vi "MH.vi"() -> ()   [LabVIEW 2018]
uses:
  <vilib>/Utility/file.llb/Read Delimited Spreadsheet (DBL).vi
panel:
  in  "stop":bool
  in  "Main Tab Control":T1(tab)
  in  "?":bool
  in  "MH data folder:":path=path "C:/Research/data/MH"
  out "File path for today's data":path
  in  "Short comment on today's measurement (will be the info file filename)":string="todayssample"
  in  "Long comment on today's measurement":string="This is where you can put more information about this measurement."
  in  "ImpedanceGFactor Tab Control":enum32{"H-Coil", "M- Coil"}(tab)
  in  "H-Coil Tab Control":T2(tab)
  in  "H-Coil VNA Control Tab Control":enum32{"Control Panel", "Display Panel"}(tab)
  out "isFileWritten? 2":string
  out "writeImpeadanceDataError 2":errorcluster
  in  "writeImpeadanceDataFunctionName":string
  out "Data file: data 3":dbl[][](array[numeric])
  in  "vnaEndFreq":dbl=30000000.0
  in  "vnaStartFreq":dbl=100000.0
  in  "vnaNumOfRecordings":dbl=5001.0
  in  "vnaFunctionName":string="vnaRead"
  in  "vnaRead":path=path "C:/Research/MH program/tempsScopeAndVNALabview.py"
  in  "H coil impedance data source:":enum32{"Measure:", "From data file:"}(radio)
  in  "Path: Hcoil data 2":path=path "C:/Research/data/RohdeZND/20180620/20180620-Hcoil.csv"
  in  "?":bool
  out "Data file: data 2":dbl[][](array[numeric])
  out "vnaErrorOut":errorcluster
  out "Impedance (Magnitude)":cluster{dbl[], dbl[]}(graph)
  out "Impedance (Phase)":cluster{dbl[], dbl[]}(graph)
  in  "H-Coil Manual Fit Control Tab Control":enum32{"Control Tab", "Display Tab"}(tab)
  in  "numf 1H":i16=1000
  in  "fmax 1H":dbl=20000000.0
  in  "f0 1H":dbl=1.0
  in  "Num of components in BNC model 1H":i16=10
  in  "Input: BNC cable length (ft) 1H":dbl=4.0 format="%#_6f"
  in  "Input: R2 (Ohms) 1H":dbl=10.0 format="%#_6f"
  in  "Input: R1 (Ohms) 1H":dbl=14.6 format="%#_6f"
  in  "Input: L (nH) 1H":dbl=3000.0 format="%#_6f"
  in  "Input: C (pF) 1H":dbl=60.0 format="%#_6f"
  in  "Input: C (pF) 2H":dbl=70.0 format="%#_6f"
  in  "Input: L (nH) 2H":dbl=800.0 format="%#_6f"
  in  "Input: R1 (Ohms) 2H":dbl=11.0 format="%#_6f"
  in  "Input: R2 (Ohms) 2H":dbl=25.0 format="%#_6f"
  in  "Input: BNC cable length (ft) 2H":dbl=4.0 format="%#_6f"
  in  "Num of components in BNC model 2H":i16=4
  in  "f0 2H":dbl=1.0
  in  "fmax 2H":dbl=40000000.0
  in  "numf 2H":i16=1000
  in  "?":bool
  out "Simulation 2: error out 2":errorcluster
  out "Simulation 1: error out":errorcluster
  out "Simulation 1: data":dbl[][](array[numeric]) format="%#_6f"
  out "Simulation 2: data":dbl[][](array[numeric]) format="%#_6f"
  in  "module path":path=path "C:/Research/MH program/impedancesim.py"
  in  "function name":string="impedance"
  out "?":string
  out "?":string
  out "?":string
  in  "?":bool
  in  "?":bool
  in  "?":bool=TRUE
  out "Impedance (phase)":cluster{"array":dbl[], "array":dbl[]}[](graph)
  out "Impedance (magnitude)":cluster{"array":dbl[], "array":dbl[]}[](graph)
  out "Impedance (magnitude) (zoomed)":T3(graph)
  out "Impedance (phase) (zoomed)":T3(graph)
  in  "H-Coil Automatic Fit Control Tab Control":enum32{"Control Panel", "Display Panel"}(tab)
  out "fit parameters":dbl[](array[numeric])
  in  "Vary numlumps?\n(Choose False)":string="False"
  in  "Vary BNClen?\n(Choose False)":string="False"
  in  "Vary R2?":string="True"
  in  "Vary R1?":string="False"
  in  "Vary L?":string="True"
  in  "Vary C?":string="True"
  out "BNC length (ft) H":dbl=4.0 format="%#_6f"
  out "Num of components in BNC model fit H":i16=4
  out "R20 (Ohms) H":dbl=25.0 format="%#_6f"
  out "R10 (Ohms) H":dbl=11.0 format="%#_6f"
  out "Initial value:\nL0 (H) H":dbl=800.0 format="%#_6e"
  out "C0 (F) H":dbl=70.0 format="%#_6e"
  in  "?":bool
  out "Simulation 1: error out 3":errorcluster
  in  "module path impedance fit":path=path "C:/Research/MH program/impedancelmfitforlv.py"
  in  "function name impedance fit":string="impedancelmfit"
  out "return value gH 2":dbl[][](array[numeric])
  out "cluster":T4
  out "Impedance data":cluster{dbl[], dbl[], dbl[]}
  in  "Start data pt":i32=2
  out "Total data points":i32
  in  "End data point":i32=3000
  out "Impedance mag near zero:\nFit vs data":cluster{dbl[], dbl[]}[](graph)
  out "Impedance mag data near zero: Use this to find R1":cluster{dbl[], dbl[]}(graph)
  out "?":string
  out "Impedance phase 2":T3(graph)
  out "Impedance magnitude (Ohms) 2":T3(graph)
  in  "H-Coil GFactor Control Tab Control":enum32{"Control Panel", "Display Panel"}(tab)
  in  "Coil 2":string="Hcoil"
  in  "Coil parameter source (if calculating g-factor)":enum32{"Simulation", "Fit"}(radio)=enum."Fit"
  in  "Rosc":dbl=1000000.0 format="%#_13g"
  in  "start gH":bool
  out "numf gH":i16=1000
  out "fmax gH":dbl=40000000.0
  out "f0 gH":dbl=1.0
  out "Num of components in BNC model gH":i16=4
  out "Input: BNC cable length (ft) gH":dbl=4.0 format="%#_6f"
  out "Input: R2 (Ohms) gH":dbl=25.0 format="%#_6f"
  out "Input: R1 (Ohms) gH":dbl=11.0 format="%#_6f"
  out "Input: L (H) gH":dbl=800.0 format="%#_6f"
  out "Input: C (F) gH":dbl=70.0 format="%#_6f"
  out "numf gH 2":i16=1000
  out "fmax gH 2":dbl=40000000.0
  out "f0 gH 2":dbl=1.0
  out "Num of components in BNC model gH 2":i16=4
  out "Input: BNC cable length (ft) gH 2":dbl=4.0 format="%#_6f"
  out "Input: R2 (Ohms) gH 2":dbl=25.0 format="%#_6f"
  out "Input: R1 (Ohms) gH 2":dbl=11.0 format="%#_6f"
  out "Input: L (H) gH 2":dbl=800.0 format="%#_6f"
  out "Input: C (F) gH 2":dbl=70.0 format="%#_6f"
  in  "G-Factor Calculation":T5(radio)
  in  "Date 3":string
  in  "Time 3":string
  in  "Filepath Name":string="C:/Research/Data/MH"
  out "readG-FactorFilesError":errorcluster
  in  "ReadDataFunctionName":string="readGFactorData"
  out "Simulation 1: error out 2":errorcluster
  out "return value gH":dbl[][](array[numeric])
  in  "function name gfactor":string="gfactor"
  in  "module path g-factor":path=path "C:/Research/MH program/gfactor.py"
  out "gfactor H (phase)":T6(graph)
  out "gfactor H (magnitude)":T6(graph)
  in  "M-Coil Control Tab Control":T7(tab)
  in  "M-Coil VNA Control Tab Control":enum32{"Control Panel", "Display Panel"}(tab)
  in  "writeImpeadanceDataFunctionName 2":string
  out "writeImpeadanceDataError":errorcluster
  out "isFileWritten?":string
  out "Data file: data 4":dbl[][](array[numeric])
  out "Data file: M coil data":dbl[][](array[numeric])
  in  "Path: Mcoil data":path=path "C:/Research/data/RohdeZND/20180621/20180621-Mcoil.csv"
  out "error out":errorcluster
  in  "M coil impedance data source:":enum32{"Measure:", "From data file:"}(radio)
  in  "?":bool
  in  "vnaRead 2":path=path "C:/Research/MH program/tempsScopeAndVNALabview.py"
  in  "vnaFunctionName 2":string="vnaRead"
  in  "vnaNumOfRecordings 2":dbl=5001.0
  in  "vnaStartFreq 2":dbl=100000.0
  in  "vnaEndFreq 2":dbl=30000000.0
  out "M Impedance (Phase)":cluster{dbl[], dbl[]}(graph)
  out "M Impedance (Magnitude)":cluster{dbl[], dbl[]}(graph)
  in  "M-Coil Manual Fit Control Tab Control":enum32{"Control Panel", "Display Panel"}(tab)
  in  "numf 1M":i16=1000
  in  "fmax 1M":dbl=40000000.0
  in  "f0 1M":dbl=1.0
  in  "Num of components in BNC model 1M":i16=10
  in  "Input: BNC cable length (ft) 1M":dbl=4.0 format="%#_6f"
  in  "Input: R2 (Ohms) 1M":dbl=14.5 format="%#_6f"
  in  "Input: R1 (Ohms) 1M":dbl=8.05 format="%#_6f"
  in  "Input: L (nH) 1M":dbl=1400.0 format="%#_6f"
  in  "Input: C (pF) 1M":dbl=64.0 format="%#_6f"
  in  "Input: C (pF) 2M":dbl=70.0 format="%#_6f"
  in  "Input: L (nH) 2M":dbl=800.0 format="%#_6f"
  in  "Input: R1 (Ohms) 2M":dbl=11.0 format="%#_6f"
  in  "Input: R2 (Ohms) 2M":dbl=25.0 format="%#_6f"
  in  "Input: BNC cable length (ft) 2M":dbl=4.0 format="%#_6f"
  in  "Num of components in BNC model 2M":i16=4
  in  "f0 2M":dbl=1.0
  in  "fmax 2M":dbl=40000000.0
  in  "numf 2M":i16=1000
  in  "python impedance":path=path "C:/Research/MH program/impedancesim.py"
  in  "python impedance function name":string="impedance"
  in  "?":bool
  out "Simulation 2M: data":dbl[][](array[numeric]) format="%#_6f"
  out "Simulation 1M: data":dbl[][](array[numeric]) format="%#_6f"
  out "Simulation 1M: error out":errorcluster
  out "Simulation 2M: error out":errorcluster
  out "?":string
  out "?":string
  out "?":string
  in  "?":bool
  in  "?":bool
  in  "?":bool=TRUE
  out "Impedance (phase) M":cluster{"array":dbl[], "array":dbl[]}[](graph)
  out "Impedance (magnitude) M":cluster{"array":dbl[], "array":dbl[]}[](graph)
  out "Impedance (magnitude) M (zoomed)":T3(graph)
  out "Impedance (phase) M (zoomed)":T3(graph)
  in  "M-Coil Automatic Fit Control Tab Control":enum32{"Control Panel", "Display Panel"}(tab)
  out "C0 (F) H 2":dbl=70.0 format="%#_6e"
  out "Initial value:\nL0 (H) H 2":dbl=800.0 format="%#_6e"
  out "R10 (Ohms) H 2":dbl=11.0 format="%#_6f"
  out "R20 (Ohms) H 2":dbl=25.0 format="%#_6f"
  out "Num of components in BNC model fit H 2":i16=4
  out "BNC length (ft) H 2":dbl=4.0 format="%#_6f"
  in  "Vary C? 2":string="True"
  in  "Vary L? 2":string="True"
  in  "Vary R1? 2":string="False"
  in  "Vary R2? 2":string="True"
  in  "Vary BNClen?\n(Choose False) 2":string="False"
  in  "Vary numlumps?\n(Choose False) 2":string="False"
  in  "?":bool
  in  "End data point 2":i32=3000
  out "Total data points 2":i32
  out "Impedance data 2":cluster{dbl[], dbl[], dbl[]}
  in  "Start data pt 2":i32=2
  out "Simulation 1: error out 4":errorcluster
  in  "module path impedance fit 2":path=path "C:/Research/MH program/impedancelmfitforlv.py"
  in  "function name impedance fit 2":string="impedancelmfit"
  out "return value":dbl[][](array[numeric])
  out "fit parameters 2":dbl[](array[numeric])
  out "cluster 2":T4
  out "Impedance magnitude (Ohms)":T3(graph)
  out "Impedance phase":T3(graph)
  out "Impedance mag near zero:\nFit vs data 2":cluster{dbl[], dbl[]}[](graph)
  out "Impedance mag near zero: Use this to find R1":cluster{dbl[], dbl[]}(graph)
  in  "M-Coil GFactor Control Tab Control":enum32{"Control Panel", "Display Panel"}(tab)
  in  "Coil":string="Mcoil"
  in  "Filepath Name 2":string="C:/Research/Data/MH"
  in  "Time 2":string
  in  "Date 2":string
  in  "Rosc 2":dbl=1000000.0 format="%#_13g"
  in  "G-Factor Calculation 2":T5(radio)
  in  "Coil parameter source":enum32{"Simulation", "Fit"}(radio)=enum."Fit"
  in  "start gM":bool
  out "Input: C (F) gM":dbl=70.0 format="%#_6f"
  out "Input: L (H) gM":dbl=800.0 format="%#_6f"
  out "Input: R1 (Ohms) gM":dbl=11.0 format="%#_6f"
  out "Input: R2 (Ohms) gM":dbl=25.0 format="%#_6f"
  out "Num of components in BNC model gM":i16=4
  out "Input: BNC cable length (ft) gM":dbl=4.0 format="%#_6f"
  out "f0 gM":dbl=1.0
  out "fmax gM":dbl=40000000.0
  out "numf gM":i16=1000
  out "numf gM 2":i16=1000
  out "fmax gM 2":dbl=40000000.0
  out "f0 gM 2":dbl=1.0
  out "Num of components in BNC model gM 2":i16=4
  out "Input: BNC cable length (ft) gM 2":dbl=4.0 format="%#_6f"
  out "Input: R2 (Ohms) gM 2":dbl=25.0 format="%#_6f"
  out "Input: R1 (Ohms) gM 2":dbl=11.0 format="%#_6f"
  out "Input: L (H) gM 2":dbl=800.0 format="%#_6f"
  out "Input: C (F) gM 2":dbl=70.0 format="%#_6f"
  in  "ReadDataFunctionName 2":string="readGFactorData"
  in  "module path g-factor 2":path=path "C:/Research/MH program/gfactor.py"
  in  "function name gfactor 2":string="gfactor"
  out "readG-FactorFilesError  2":errorcluster
  out "gfactor M: error out":errorcluster
  out "return value gM":dbl[][](array[numeric])
  out "gfactor M (magnitude)":T6(graph)
  out "gfactor M (phase)":T6(graph)
  in  "VoltageTemp Control Tab Control":enum32{"Control Panel", "Display Panel"}(tab)
  in  "Run with Simulator":bool=TRUE
  in  "Run":i64
  in  "Run":dbl
  in  "readDataFileVoltageName":string="readVoltageData"
  in  "Voltage data source:":enum32{"Measure:", "From data file:"}(radio)
  in  "readDataFileTemperatureName":string="readTempData"
  in  "Date":string
  in  "Time":string
  in  "numChan 2":i32=2
  in  "dataFilePath":string="C:\\Research\\data\\MH"
  in  "?":bool
  in  "numChan":i32=2
  in  "scopeNumCollects":i32=3
  in  "shortRecordLength":i32=10000
  in  "longRecordLength 2":i32=100000
  in  "mainForAmbrell":string="mainForAmbrell"
  in  "ModulePath":path=path "C:/Research/SenaCodeBaseandDocuments/CodeBaseRepo/SummerResearch2019CodeBase/MH program/tempsScopeAndVNALabviewMHProgram.py"
  in  "Operating Frequency of EASYHEAT":dbl=227000.0
  in  "Run Checkscale?":bool=TRUE
  out "readDataFileTempError":errorcluster
  out "readDataFileVoltageError":errorcluster
  out "mainForAmbrellError":errorcluster
  out "Oscilloscope Channel 1 Output Graph":cluster{dbl[], dbl[]}[](graph)
  out "Oscilloscope Channel 2 Output Graph":cluster{dbl[], dbl[]}[](graph)
  out "Opsens Channel 1":cluster{"Array 2":dbl[], "Array 3":dbl[]}[](graph)
  # "Instructions for making an M(H) measurement"
  # "0. (Rarely) Calibrate H (still need to work on this)\n1. (Sometimes) Measure impedance of H coil using vector network analyzer (Sena's program) or load from file\n2. (Sometimes) Model impedance of H coil to find coil parameters (Zoe's program)\n3. (Sometimes) Calculate g-factor of H coil (Zoe's program)\n4. (Sometimes) Measure impedance of M coil using vector network analyzer (Sena's program) or load from file\n5. (Sometimes) Model impedance of M coil to find coil parameters (Zoe's program)\n6. (Sometimes) Calculate g-factor of M coil (Zoe's program)\n7. (Every time) Center M coil by hand (no program)\n8. (Every time) Measure sample data - induced voltage using oscilloscope and temperature using opsens (Sena's program) or load from file(s)\n9. (Every time) Select voltage data to analyze (Emily's program)\n10. (Every time) Analyze voltage data to find M(H) for each run (Emily's program)\n11. (Every time) Save data (Emily's program)"
  # "CONNECT M COIL TO VNA!"
  # "H coil"
  # "Impedance\nsimulation 1\nparameters"
  # "Impedance\nsimulation 2\nparameters"
  # "Data file\nlocation"
  # "What to plot:"
  # "(toggle buttons below)"
  # "Simulation 1"
  # "Simulation 2"
  # "Data file"
  # "Values to initialize fit:"
  # "THIS MAY TAKE A\nCOUPLE MINUTES!"
  # "f"
  # "Z (mag)"
  # "Z (phase)"
  # "H coil"
  # "Calculate g-factor"
  # "Oscillosope\nimpedance:"
  # "THIS MAY TAKE A\nCOUPLE MINUTES!"
  # "Read Data File Controls"
  # "Impedance\nsimulation 1\nparameters"
  # "Fit\nparameters"
  # "CONNECT H COIL TO VNA!"
  # "M coil"
  # "Impedance\nsimulation 1\nparameters"
  # "Impedance\nsimulation 2\nparameters"
  # "Data file\nlocation"
  # "What to plot:"
  # "(toggle buttons below)"
  # "Simulation 1"
  # "Simulation 2"
  # "Data file"
  # "THIS MAY TAKE A\nCOUPLE MINUTES!"
  # "Read Data File Controls"
  # "M coil"
  # "Calculate g-factor"
  # "THIS MAY TAKE A\nCOUPLE MINUTES!"
  # "Oscillosope\nimpedance:"
  # "Impedance\nsimulation 1\nparameters"
  # "(Imported from\n last panel)"
  # "(Currently not working - need to decide on a data format)"
  # "Save data to an Excel file. Use multiple worksheets within one file to store the various types of data. e.g.\n-One worksheet to store basic info about the data collection and analysis:\n       -Date and time\n       -Calibration factors\n-One worksheet to store the Hcoil impedance\n       -Headers: Frequency (Hz) // Real component (Ohms) // Imag component (Ohms) // Note: Data from file or measured?\n       -freq, real, imag columns\n-One worksheet to store info on the Hcoil impedance model\n       -Was the impedance model the result of a manual fit (simulation) or an automatic fit?\n       -If automatic fit, which parameters were allowed to vary, and which were kept fixed?\n       -Values for C, L, R1, R2, BNClen, numlumps\n-One worksheet for Hcoil impedance model, similar to data\n       -Headers: Frequency (Hz) // Real component (Ohms) // Imag component (Ohms)\n       -freq, real, imag columns\n-One sheet showing a chart of impedance data vs model\n-One worksheet for Hcoil gfactor\n       -Headers: Frequency (Hz) // Real component  // Imag component \n       -freq, real, imag columns\n-One sheet showing a chart of Hcoil gfactor\n-Same series of sheets as above but for Mcoil\n-One worksheet to store basic info about the voltage/temperature data collection and analysis\n       -How many data collections? Record length?\n       -Time data collection was begun\n       -Info about temperature collection - time between data points?\n-One worksheet for EACH set of voltage data\n-One worksheet for temperature vs time data\n-One worksheet for all the M(H) curves analyzed\n-One sheet at the end showing a chart of M(H) for all data sets\n\n\nOpen question:\nIs it a good idea to do all this in Excel?? We could run into problems with memory for large Excel files. If Excel is a problem, a series of .txt or .csv files (one for each sheet above) could accomplish the same goals.\nIf we do it this way, we should create organized folders for each analysis."
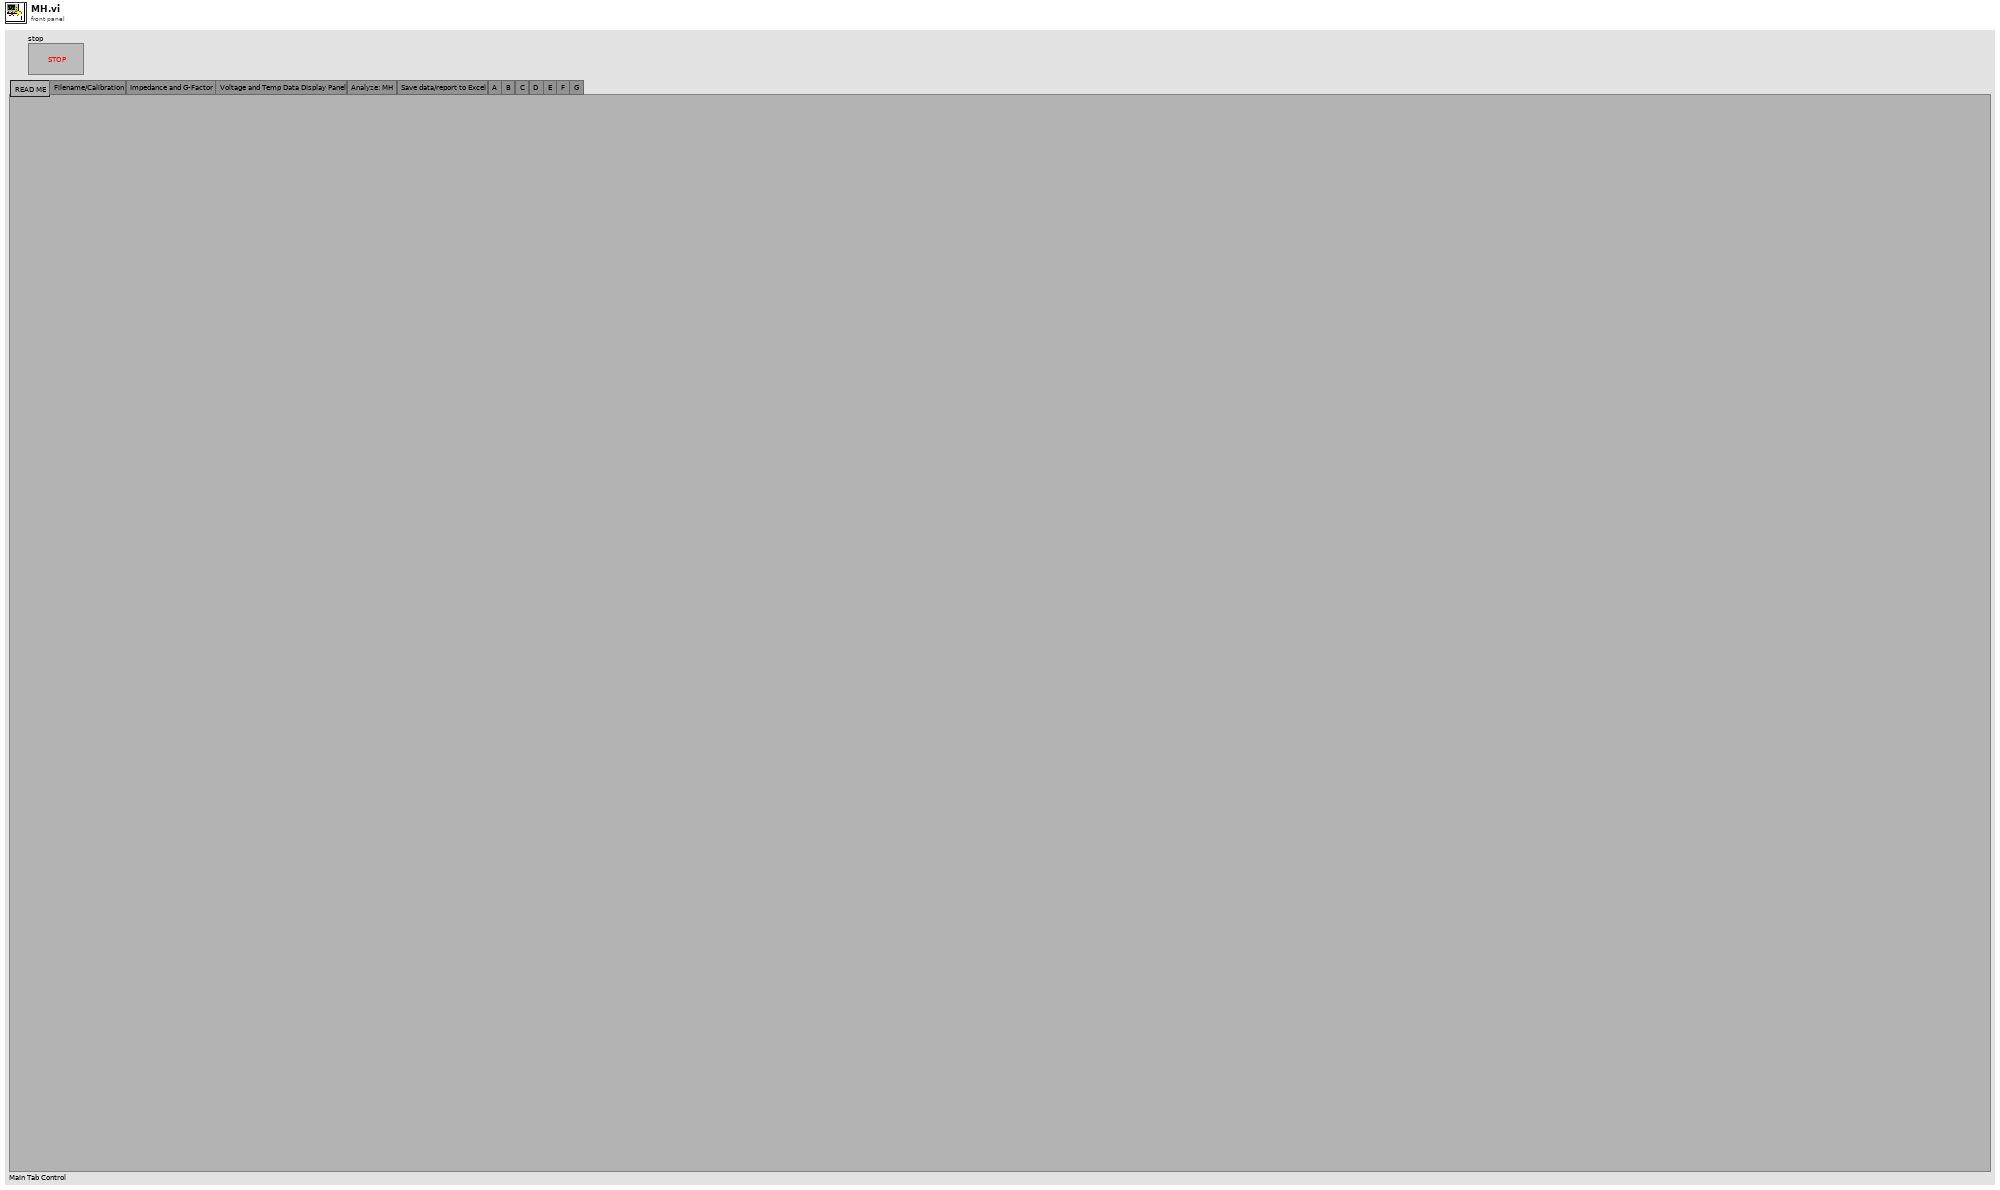
[diagram p1: front panel]
types:
  T1 = enum32{"READ ME", "Filename/Calibration", "Impedance and G-Factor", "Voltage and Temp Data Display Panel", "Analyze: MH", "Save data/report to Excel", "A", "B", "C", "D", "E", "F", "G"}
  T2 = enum32{"Get Impedance from VNA", "Manual Fit H-Coil", "Automatic Fit H-Coil", "G-Factor Calculation"}
  T3 = cluster{"return value 3":dbl[], "return value 3":dbl[]}[]
  T4 = cluster{"[0]":dbl, "[1]":dbl, "[2]":dbl, "[3]":dbl, "[4]":dbl, "[5]":dbl, "[6]":dbl, "[7]":dbl, "[8]":dbl}
  T5 = enum32{"Read data from a g-factor file", "Calculate G-factor"}
  T6 = cluster{"return value 3":dbl[], "return value 3":dbl[]}
  T7 = enum32{"Get Impedance from VNA", "Manual Fit M-Coil", "Automatic Fit M-Coil", "G-Factor Calculation"}
  T8 = cluster{dbl, dbl, "Input: R1 (Ohms) 1H":dbl, "Input: R2 (Ohms) 1H":dbl, "Input: BNC cable length (ft) 1H":dbl, "Num of components in BNC model 1H":i16, "f0 1H":dbl, "fmax 1H":dbl, "numf 1H":i16}
  T9 = cluster{dbl, dbl, "Input: R1 (Ohms) 2H":dbl, "Input: R2 (Ohms) 2H":dbl, "Input: BNC cable length (ft) 2H":dbl, "Num of components in BNC model 2H":i16, "f0 2H":dbl, "fmax 2H":dbl, "numf 2H":i16}
  T10 = cluster{dbl, dbl, "Input: R1 (Ohms) 2M":dbl, "Input: R2 (Ohms) 2M":dbl, "Input: BNC cable length (ft) 2M":dbl, "Num of components in BNC model 2M":i16, "f0 2M":dbl, "fmax 2M":dbl, "numf 2M":i16}
  T11 = cluster{dbl, dbl, "Input: R1 (Ohms) 1M":dbl, "Input: R2 (Ohms) 1M":dbl, "Input: BNC cable length (ft) 1M":dbl, "Num of components in BNC model 1M":i16, "f0 1M":dbl, "fmax 1M":dbl, "numf 1M":i16}
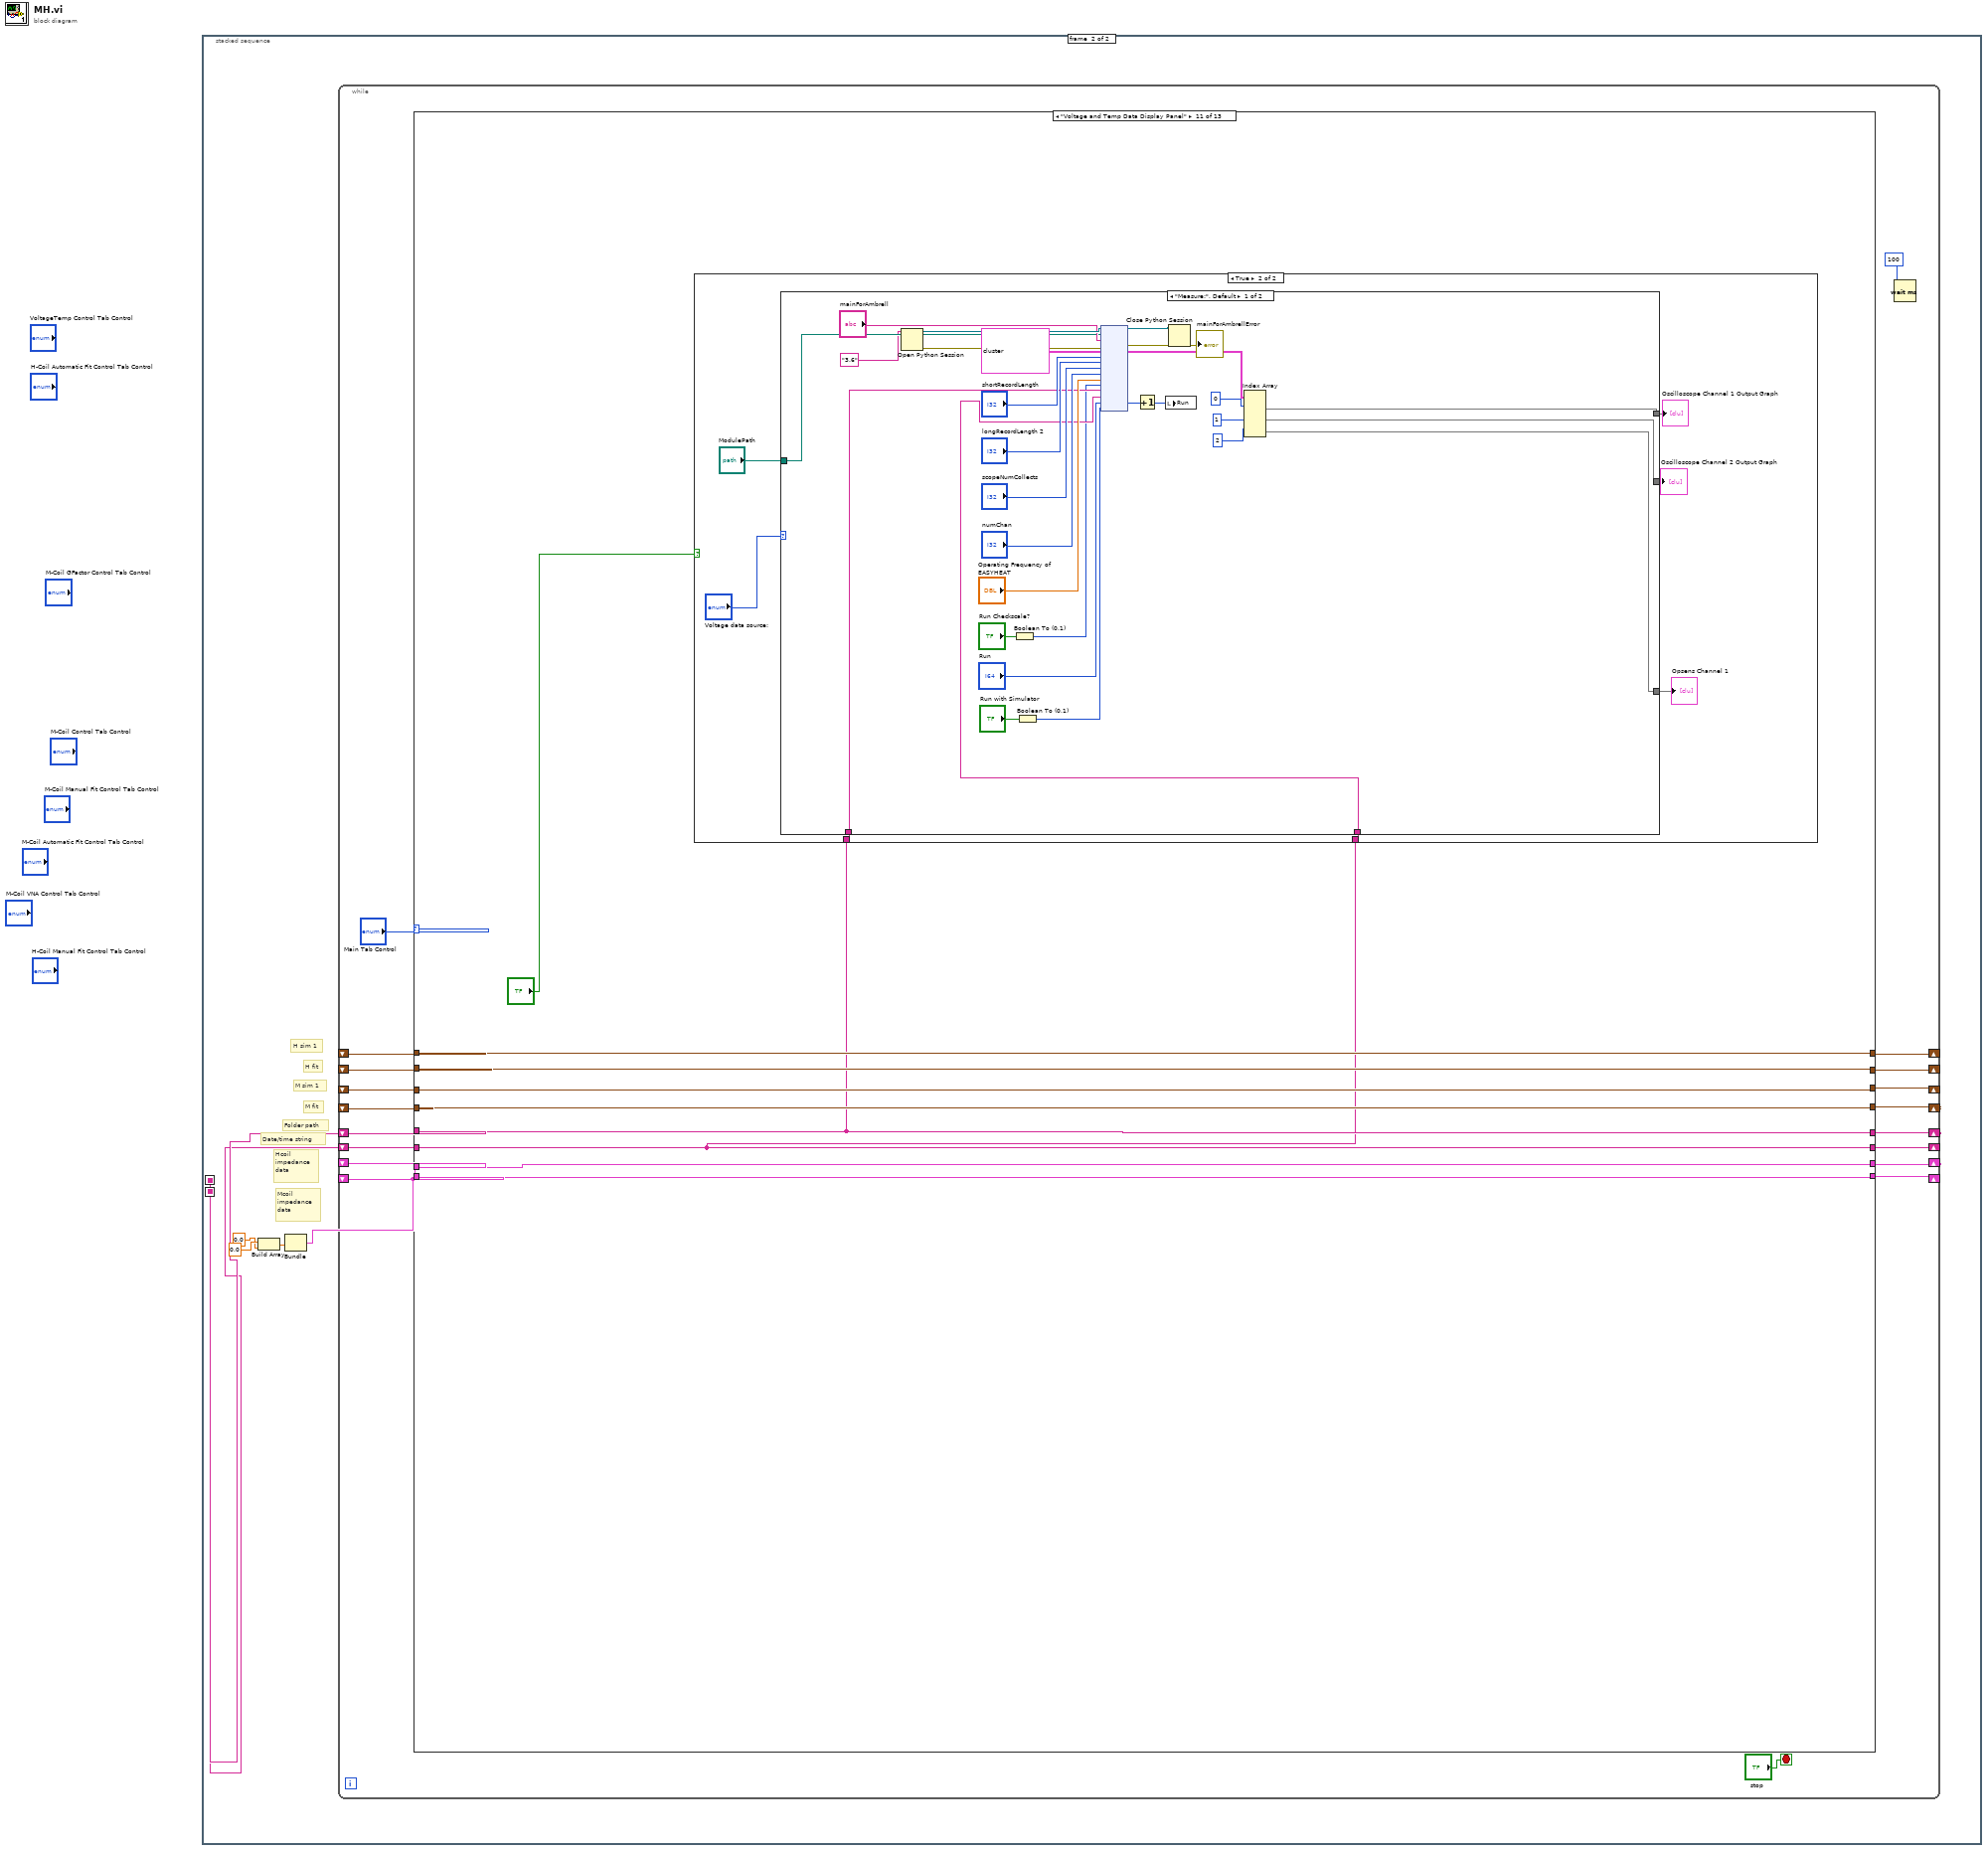
[diagram p0: block diagram]
diagram:
  n1 = stacked-sequence {
    seq-local: [w2 _] -> [_ w36]
    seq-local: [w1 _] -> [_ w35]
    frame #0 {
      n2 = stacked-sequence {
        seq-local: [w3 _ _] -> [_ w12 w14]
        tunnel: [_ w12 _] -> w2
        tunnel: [w4 _ _] -> w1
        frame #0 {
          w7 = "\\\\"
          n3 = Format Date/Time String(time format string (%c)="%Y%m%d") -> (date/time string=w6:string)  [unwired: 2 in]
          n4 = Format Date/Time String(time format string (%c)="%H%M%S") -> (date/time string=w5:string)  [unwired: 2 in]
          n5 = Path To String(path="MH data folder:") -> (string=w9:string)
          n6 = Concatenate Strings(w9, w7, w6, w7, w5) -> (w3:string)
          n7 = Concatenate Strings(w6, w5) -> (w4:string)
        }
        frame #1 {
          n8 = String To Path(string=w12) -> (path=w13:path)
          "File path for today's data" <- w13
          n9 = Create Folder(path (use dialog)=w13) -> ()  [unwired: 2 in, 3 out]
        }
        frame #2 {
          n10 = Concatenate Strings(w14, "\\\\", "Oscilloscope") -> (w25:string)
          n11 = Concatenate Strings(w14, "\\\\", "Opsens") -> (w21:string)
          n12 = Concatenate Strings(w14, "\\\\", "MHanalyzed") -> (w17:string)
          n13 = Concatenate Strings(w14, "\\\\", "Mcoil") -> (w29:string)
          n14 = Concatenate Strings(w14, "\\\\", "Hcoil") -> (w32:string)
          n15 = String To Path(string=w25) -> (path=w23:path)
          n16 = String To Path(string=w21) -> (path=w19:path)
          n17 = String To Path(string=w17) -> (path=w15:path)
          n18 = String To Path(string=w29) -> (path=w28:path)
          n19 = String To Path(string=w32) -> (path=w31:path)
          n20 = Create Folder(path (use dialog)=w23) -> ()  [unwired: 2 in, 3 out]
          n21 = Create Folder(path (use dialog)=w19) -> ()  [unwired: 2 in, 3 out]
          n22 = Create Folder(path (use dialog)=w15) -> ()  [unwired: 2 in, 3 out]
          n23 = Create Folder(path (use dialog)=w28) -> ()  [unwired: 2 in, 3 out]
          n24 = Create Folder(path (use dialog)=w31) -> ()  [unwired: 2 in, 3 out]
        }
      }
    }
    frame #1 {
      # "Date/time string"
      # "Folder path"
      # "H sim 1"
      # "H fit"
      # "M sim 1"
      # "M fit"
      # "Hcoil\nimpedance\ndata"
      # "Mcoil\nimpedance\ndata"
      n25 = Build Array(0.0, 0.0) -> (w37:dbl[])
      n26 = Bundle(w37, w37, w37) -> (w38:cluster{dbl[], dbl[], dbl[]})  [unwired: 1 in]
      n27 = while {
        shift-right: [w57] -> _
        shift-left: _ -> [w56]
        shift-right: [w55] -> _
        shift-left: _ -> [w54]
        shift-right: [w52] -> _
        shift-left: w38 -> [w53]
        shift-right: [w51] -> _
        shift-left: w38 -> [w50]
        shift-right: [w49] -> _
        shift-left: _ -> [w48]
        shift-right: [w47] -> _
        shift-left: _ -> [w46]
        shift-right: [w45] -> _
        shift-left: w36 -> [w44]
        shift-right: [w41] -> _
        shift-left: w35 -> [w42]
        stop <- "stop" stop-if-true
        n28 = case shown="\"Voltage and Temp Data Display Panel\"" "Main Tab Control" {
          tunnel: [w67 w74 w93 w203 w412 w477 w624 w710 w920 w986 w1129 w1222 w1232] -> w57
          tunnel: w56 -> [w67 w74 w93 _ w412 w477 w624 w710 w920 w986 w1129 w1222 w1232]
          tunnel: [w66 w73 w92 w201 w411 w476 w623 w711 w917 w981 w1127 w1221 w1230] -> w55
          tunnel: w54 -> [w66 w73 w92 w201 w411 w476 w623 _ w917 w981 w1127 w1221 w1230]
          tunnel: w53 -> [w65 w76 w87 w199 w410 w475 w625 w708 w916 w985 w1125 w1224 w1228]
          tunnel: [w65 w76 w84 w199 w410 w475 w625 w708 w916 w985 w1125 w1224 w1228] -> w52
          tunnel: [w64 w75 w91 w198 w409 w474 w626 w707 w918 w984 w1124 w1223 w1227] -> w51
          tunnel: w50 -> [w64 w75 w91 w198 w409 w474 w620 w707 w918 w984 w1124 w1223 w1227]
          tunnel: [w63 w72 w90 w197 w407 w473 w622 w706 w919 w983 w1128 w1220 w1231] -> w49
          tunnel: w48 -> [w63 w72 w90 w197 w380 w473 w622 w706 w919 w983 w1128 w1220 w1231]
          tunnel: [w62 w71 w89 w196 w406 w472 w621 w705 w915 w980 w1126 w1219 w1229] -> w47
          tunnel: w46 -> [w62 w71 w89 w196 w406 w472 w621 w705 w893 w980 w1126 w1219 w1229]
          tunnel: [w61 w70 w86 w195 w381 w471 w617 w704 w889 w979 w1122 w1218 w1226] -> w45
          tunnel: w44 -> [w61 w70 w86 w195 w381 w471 w617 w704 w889 w979 w1122 w1218 w1226]
          tunnel: w42 -> [w60 w68 w85 w194 w384 w470 w616 w703 w892 w978 w1121 w1217 w1225]
          tunnel: [w60 w68 w85 w194 w384 w470 w616 w703 w892 w978 w1121 w1217 w1225] -> w41
          frame "READ ME" {
          }
          frame "Filename/Calibration" {
            n29 = case shown="True" "?" {
              tunnel: w70 -> [_ w77]
              frame False {
              }
              frame True {
                n30 = String To Path(string=w77) -> (path=w78:path)
                n31 = Concatenate Strings("Short comment on today's measurement (will be the info file filename)", ".txt") -> (w81:string)
                n32 = Build Path(base path=w78, name or relative path=w81) -> (appended path=w80:path)
                n33 = Write to Text File(file (use dialog)=w80, text="Long comment on today's measurement") -> ()  [unwired: 2 in, 3 out]
              }
            }
          }
          frame "Impedance and G-Factor" {
            n34 = case shown="\"H-Coil\", Default" "ImpedanceGFactor Tab Control" {
              tunnel: w87 -> [w97 w193]
              tunnel: w86 -> [w96 _]
              tunnel: w85 -> [w95 _]
              tunnel: [w94 w193] -> w84
              frame "H-Coil", Default {
                n35 = case shown="\"Get Impedance from VNA\", Default" "H-Coil Tab Control" {
                  tunnel: w97 -> [w102 w192]
                  tunnel: w96 -> [w101 _]
                  tunnel: w95 -> [w100 _]
                  tunnel: [w99 w192] -> w94
                  frame "Get Impedance from VNA", Default {
                    n36 = case shown="\"Control Panel\", Default" "H-Coil VNA Control Tab Control" {
                      tunnel: w102 -> [w109 w191]
                      tunnel: w101 -> [w108 _]
                      tunnel: w100 -> [w107 _]
                      tunnel: [w106 w191] -> w99
                      frame "Control Panel", Default {
                        n37 = case shown="True" "?" {
                          tunnel: [w114 w118] -> w105
                          tunnel: [w111 w117] -> w104
                          tunnel: [w116 w121] -> w106
                          tunnel: w109 -> [w116 _]
                          tunnel: w108 -> [_ w120]
                          tunnel: w107 -> [_ w119]
                          frame False {
                            n38 = Unbundle(w116) -> (w113:dbl[], w115:dbl[], w112:dbl[])
                            n39 = Bundle(w113, w115) -> (w114:cluster{dbl[], dbl[]})  [unwired: 1 in]
                            n40 = Bundle(w113, w112) -> (w111:cluster{dbl[], dbl[]})  [unwired: 1 in]
                          }
                          frame True {
                            n41 = case shown="\"Measure:\", Default" "H coil impedance data source:" {
                              tunnel: [w140 w171] -> w118
                              tunnel: [w138 w170] -> w117
                              tunnel: [w141 w168] -> w121
                              tunnel: w120 -> [w132 _]
                              tunnel: w119 -> [w131 _]
                              frame "Measure:", Default {
                                n42 = Open Python Session(python version="3.6" ("Python version")) -> (session out=w155:refnum<k35>, error out=w154:errorcluster)  [unwired: 2 in]
                                n43 = Open Python Session(python version="3.6" ("Python version")) -> (session out=w135:refnum<k35>, error out=w129:errorcluster)  [unwired: 2 in]
                                n44 = node(w155, "vnaRead", "vnaFunctionName", w154, dbl[][] [], "vnaNumOfRecordings", "vnaStartFreq", "vnaEndFreq") -> (w153:refnum<k35>, w152:errorcluster, w133:dbl[][])  [unwired: 3 in, 2 out]
                                "Data file: data 3" <- w133
                                n45 = Close Python Session(session in=w153, error in=w152) -> (11:→"vnaErrorOut":errorcluster)
                                n46 = node(w135, "vnaRead", "writeImpeadanceDataFunctionName", w129, "", w133, w132, w131, "Hcoil") -> (w136:refnum<k35>, w128:errorcluster, →"isFileWritten? 2":string)  [unwired: 4 in, 2 out]
                                n47 = Index Array(array=w133, index (row) #1=0, index (row) #2=1 ("index (page)"), index (row) #3=2 ("index (page)")) -> (element #1=w139:dbl[], element #2=w150:dbl[], element #3=w149:dbl[])  [unwired: 3 in]
                                n48 = Close Python Session(session in=w136, error in=w128) -> (11:→"writeImpeadanceDataError 2":errorcluster)
                                n49 = Divide(x=w149, y=w150) -> (x/y=w148:dbl[])
                                n50 = Multiply(x=w150, y=w150) -> (x*y=w145:dbl[])
                                n51 = Inverse Tangent(1:w148) -> (0:w137:dbl[])
                                n52 = Multiply(x=w149, y=w149) -> (x*y=w146:dbl[])
                                n53 = Add(x=w145, y=w146) -> (x+y=w147:dbl[])
                                n54 = Square Root(x=w147) -> (sqrt(x)=w151:dbl[])
                                n55 = Bundle(w139, w137) -> (w138:cluster{dbl[], dbl[]})  [unwired: 1 in]
                                n56 = Bundle(w139, w151) -> (w140:cluster{dbl[], dbl[]})  [unwired: 1 in]
                                n57 = Bundle(w139, w151, w137) -> (w141:cluster{dbl[], dbl[], dbl[]})  [unwired: 1 in]
                              }
                              frame "From data file:" {
                                n58 = call-poly <vilib>:"Read Delimited Spreadsheet.vi"("file path (dialog if empty)"="Path: Hcoil data 2", "start of read offset (chars.:0)"=49, "delimiter (\\t)"="," ("delimiter (\\t)")) -> ("all rows"=w167:dbl[][])  [unwired: 7 in, 5 out]
                                n59 = Array Subset(array=w167, index (row)=1 ("index"), length (row)=10000000 ("length")) -> (w166:dbl[][])  [unwired: 2 in]
                                n60 = Transpose 2D Array(2D array=w166) -> (transposed array=w185:dbl[][])
                                "Data file: data 2" <- w185
                                n61 = Index Array(array=w185, index (row) #1=0, index (row) #2=1 ("index (page)"), index (row) #3=2 ("index (page)")) -> (element #1=w189:dbl[], element #2=w184:dbl[], element #3=w183:dbl[])  [unwired: 3 in]
                                n62 = Divide(x=w183, y=w184) -> (x/y=w182:dbl[])
                                n63 = Multiply(x=w184, y=w184) -> (x*y=w179:dbl[])
                                n64 = Inverse Tangent(1:w182) -> (0:w169:dbl[])
                                n65 = Multiply(x=w183, y=w183) -> (x*y=w180:dbl[])
                                n66 = Add(x=w179, y=w180) -> (x+y=w181:dbl[])
                                n67 = Square Root(x=w181) -> (sqrt(x)=w190:dbl[])
                                n68 = Get Date/Time String(want seconds? (F)=TRUE) -> (date string=w186:string, time string=w188:string)  [unwired: 2 in]
                                n69 = Path To String(path="Path: Hcoil data 2") -> ()  [unwired: 1 out]
                                n70 = call <vilib>:"Space Constant.vi"() -> ("String"=w187:string)
                                n71 = Bundle(w189, w169) -> (w170:cluster{dbl[], dbl[]})  [unwired: 1 in]
                                n72 = Bundle(w189, w190) -> (w171:cluster{dbl[], dbl[]})  [unwired: 1 in]
                                n73 = Bundle(w189, w190, w169) -> (w168:cluster{dbl[], dbl[], dbl[]})  [unwired: 1 in]
                                n74 = Concatenate Strings("Getting data from file...", w186, w187, w188) -> ()  [unwired: 1 out]
                              }
                            }
                          }
                        }
                        "Impedance (Magnitude)" <- w105
                        "Impedance (Phase)" <- w104
                      }
                      frame "Display Panel" {
                      }
                    }
                  }
                  frame "Manual Fit H-Coil" {
                  }
                }
              }
              frame "M- Coil" {
              }
            }
          }
          frame "A" {
            n75 = Divide(x="Input: L (nH) 2H", y=1000000000.0) -> (x/y=w222:dbl)
            n76 = Divide(x="Input: C (pF) 1H", y=1000000000000.0) -> (x/y=w210:dbl)
            n77 = Divide(x="Input: L (nH) 1H", y=1000000000.0) -> (x/y=w211:dbl)
            n78 = Divide(x="Input: C (pF) 2H", y=1000000000000.0) -> (x/y=w221:dbl)
            n79 = Bundle(w210, w211, "Input: R1 (Ohms) 1H"="Input: R1 (Ohms) 1H", "Input: R2 (Ohms) 1H"="Input: R2 (Ohms) 1H", "Input: BNC cable length (ft) 1H"="Input: BNC cable length (ft) 1H", "Num of components in BNC model 1H"="Num of components in BNC model 1H", "f0 1H"="f0 1H", "fmax 1H"="fmax 1H", "numf 1H"="numf 1H") -> (w203:T8)  [unwired: 1 in]
            n80 = Bundle(w221, w222, "Input: R1 (Ohms) 2H"="Input: R1 (Ohms) 2H", "Input: R2 (Ohms) 2H"="Input: R2 (Ohms) 2H", "Input: BNC cable length (ft) 2H"="Input: BNC cable length (ft) 2H", "Num of components in BNC model 2H"="Num of components in BNC model 2H", "f0 2H"="f0 2H", "fmax 2H"="fmax 2H", "numf 2H"="numf 2H") -> (w202:T9)  [unwired: 1 in]
            n81 = case shown="True" "?" {
              tunnel: w203 -> [_ w261]
              tunnel: w202 -> [_ w260]
              tunnel: w199 -> [_ w230]
              frame False {
              }
              frame True {
                n82 = Build Array(0.0, 0.0) -> (w247:dbl[])
                n83 = Build Array(0.0, 0.0) -> (w244:dbl[])
                n84 = Build Array(0.0, 0.0) -> (w241:dbl[])
                n85 = Build Array(0.0, 0.0) -> (w238:dbl[])
                n86 = Bundle(w247, w244) -> (w237:cluster{dbl[], dbl[]})  [unwired: 1 in]
                n87 = Bundle(w241, w238) -> (w236:cluster{dbl[], dbl[]})  [unwired: 1 in]
                n88 = stacked-sequence {
                  tunnel: [w271 _ _ _] -> w259
                  tunnel: [w270 _ _ _] -> w258
                  tunnel: "function name" -> [w269 w319 _ _]
                  tunnel: "module path" -> [w268 w318 _ _]
                  tunnel: "3.6" ("Python version") -> [w267 w317 _ _]